vi "FlexMag - 24-03-2023.vi"() -> ()   [LabVIEW 2018] (continued)
                          n13249 = Not(x=w18358) -> (.not. x?=w18359:bool)
                        }
                      }
                    }
                  }
                  frame #13 {
                    n13250 = local write "TC2_speed_coefficient_set"(TRUE ("TC1_close_loop_set")) -> ()
                  }
                  frame #14 {
                    n13251 = flat-sequence {
                      frame #0 {
                        n13252 = local read "waiting_TC"() -> (w18362:u32)
                        n13253 = Wait (ms)(milliseconds to wait=w18362) -> ()  [unwired: 1 out]
                      }
                      frame #1 {
                        n13254 = while {
                          stop <- w18363 stop-if-true
                          n13255 = local read "TC2_speed_coefficient_set"() -> (w18364:bool)
                          n13256 = Wait Until Next ms Multiple(millisecond multiple=u32 300) -> ()  [unwired: 1 out]
                          n13257 = Not(x=w18364) -> (.not. x?=w18363:bool)
                        }
                      }
                    }
                  }
                  frame #15 {
                    n13258 = local write "TC2_AO1_polarity(pos_to_neg)"(TRUE ("TC1_close_loop_set")) -> ()
                  }
                  frame #16 {
                    n13259 = flat-sequence {
                      frame #0 {
                        n13260 = local read "waiting_TC"() -> (w18367:u32)
                        n13261 = Wait (ms)(milliseconds to wait=w18367) -> ()  [unwired: 1 out]
                      }
                      frame #1 {
                        n13262 = while {
                          stop <- w18369 stop-if-true
                          n13263 = local read "TC2_AO1_polarity(pos_to_neg)"() -> (w18368:bool)
                          n13264 = Wait Until Next ms Multiple(millisecond multiple=u32 300) -> ()  [unwired: 1 out]
                          n13265 = Not(x=w18368) -> (.not. x?=w18369:bool)
                        }
                      }
                    }
                  }
                  frame #17 {
                    n13266 = local write "TC1_AO1_upper_limit_set"(TRUE ("TC1_close_loop_set")) -> ()
                  }
                  frame #18 {
                    n13267 = flat-sequence {
                      frame #0 {
                        n13268 = local read "waiting_TC"() -> (w18372:u32)
                        n13269 = Wait (ms)(milliseconds to wait=w18372) -> ()  [unwired: 1 out]
                      }
                      frame #1 {
                        n13270 = while {
                          stop <- w18373 stop-if-true
                          n13271 = local read "TC1_AO1_upper_limit_set"() -> (w18374:bool)
                          n13272 = Wait Until Next ms Multiple(millisecond multiple=u32 300) -> ()  [unwired: 1 out]
                          n13273 = Not(x=w18374) -> (.not. x?=w18373:bool)
                        }
                      }
                    }
                  }
                  frame #19 {
                    n13274 = local write "TC1_AO1_bottom_limit_set"(TRUE ("TC1_close_loop_set")) -> ()
                  }
                  frame #20 {
                    n13275 = flat-sequence {
                      frame #0 {
                        n13276 = local read "waiting_TC"() -> (w18377:u32)
                        n13277 = Wait (ms)(milliseconds to wait=w18377) -> ()  [unwired: 1 out]
                      }
                      frame #1 {
                        n13278 = while {
                          stop <- w18379 stop-if-true
                          n13279 = local read "TC1_AO1_bottom_limit_set"() -> (w18378:bool)
                          n13280 = Wait Until Next ms Multiple(millisecond multiple=u32 300) -> ()  [unwired: 1 out]
                          n13281 = Not(x=w18378) -> (.not. x?=w18379:bool)
                        }
                      }
                    }
                  }
                  frame #21 {
                    n13282 = local write "TC2_AO1_upper_limit_set"(TRUE ("TC1_close_loop_set")) -> ()
                  }
                  frame #22 {
                    n13283 = flat-sequence {
                      frame #0 {
                        n13284 = local read "waiting_TC"() -> (w18382:u32)
                        n13285 = Wait (ms)(milliseconds to wait=w18382) -> ()  [unwired: 1 out]
                      }
                      frame #1 {
                        n13286 = while {
                          stop <- w18383 stop-if-true
                          n13287 = local read "TC2_AO1_upper_limit_set"() -> (w18384:bool)
                          n13288 = Wait Until Next ms Multiple(millisecond multiple=u32 300) -> ()  [unwired: 1 out]
                          n13289 = Not(x=w18384) -> (.not. x?=w18383:bool)
                        }
                      }
                    }
                  }
                  frame #23 {
                    n13290 = local write "TC2_AO1_bottom_limit_set"(TRUE ("TC1_close_loop_set")) -> ()
                  }
                  frame #24 {
                    n13291 = flat-sequence {
                      frame #0 {
                        n13292 = local read "waiting_TC"() -> (w18387:u32)
                        n13293 = Wait (ms)(milliseconds to wait=w18387) -> ()  [unwired: 1 out]
                      }
                      frame #1 {
                        n13294 = while {
                          stop <- w18389 stop-if-true
                          n13295 = local read "TC2_AO1_bottom_limit_set"() -> (w18388:bool)
                          n13296 = Wait Until Next ms Multiple(millisecond multiple=u32 300) -> ()  [unwired: 1 out]
                          n13297 = Not(x=w18388) -> (.not. x?=w18389:bool)
                        }
                      }
                    }
                  }
                  frame #25 {
                    n13298 = local write "TC1_regulation_type_selection"(TRUE ("TC1_regulation_type_selection")) -> ()
                  }
                  frame #26 {
                    n13299 = flat-sequence {
                      frame #0 {
                        n13300 = local read "waiting_TC"() -> (w18392:u32)
                        n13301 = Wait (ms)(milliseconds to wait=w18392) -> ()  [unwired: 1 out]
                      }
                      frame #1 {
                        n13302 = while {
                          stop <- w18393 stop-if-true
                          n13303 = local read "TC1_regulation_type_selection"() -> (w18394:bool)
                          n13304 = Wait Until Next ms Multiple(millisecond multiple=u32 300) -> ()  [unwired: 1 out]
                          n13305 = Not(x=w18394) -> (.not. x?=w18393:bool)
                        }
                      }
                    }
                  }
                  frame #27 {
                    n13306 = local write "TC2_regulation_type_selection"(TRUE ("TC2_regulation_type_selection")) -> ()
                  }
                  frame #28 {
                    n13307 = flat-sequence {
                      frame #0 {
                        n13308 = local read "waiting_TC"() -> (w18397:u32)
                        n13309 = Wait (ms)(milliseconds to wait=w18397) -> ()  [unwired: 1 out]
                      }
                      frame #1 {
                        n13310 = while {
                          stop <- w18399 stop-if-true
                          n13311 = local read "TC2_regulation_type_selection"() -> (w18398:bool)
                          n13312 = Wait Until Next ms Multiple(millisecond multiple=u32 300) -> ()  [unwired: 1 out]
                          n13313 = Not(x=w18398) -> (.not. x?=w18399:bool)
                        }
                      }
                    }
                  }
                  frame #29 {
                    n13314 = local write "TC2_setpoint_type"(TRUE ("TC2_setpoint_type")) -> ()
                  }
                  frame #30 {
                    n13315 = flat-sequence {
                      frame #0 {
                        n13316 = local read "waiting_TC"() -> (w18402:u32)
                        n13317 = Wait (ms)(milliseconds to wait=w18402) -> ()  [unwired: 1 out]
                      }
                      frame #1 {
                        n13318 = while {
                          stop <- w18403 stop-if-true
                          n13319 = local read "TC2_setpoint_type"() -> (w18404:bool)
                          n13320 = Wait Until Next ms Multiple(millisecond multiple=u32 300) -> ()  [unwired: 1 out]
                          n13321 = Not(x=w18404) -> (.not. x?=w18403:bool)
                        }
                      }
                    }
                  }
                  frame #31 {
                    n13322 = local write "TC1_setpoint_type"(TRUE ("TC1_setpoint_type")) -> ()
                  }
                  frame #32 {
                    n13323 = flat-sequence {
                      frame #0 {
                        n13324 = local read "waiting_TC"() -> (w18407:u32)
                        n13325 = Wait (ms)(milliseconds to wait=w18407) -> ()  [unwired: 1 out]
                      }
                      frame #1 {
                        n13326 = while {
                          stop <- w18409 stop-if-true
                          n13327 = local read "TC1_setpoint_type"() -> (w18408:bool)
                          n13328 = Wait Until Next ms Multiple(millisecond multiple=u32 300) -> ()  [unwired: 1 out]
                          n13329 = Not(x=w18408) -> (.not. x?=w18409:bool)
                        }
                      }
                    }
                  }
                  frame #33 {
                    n13330 = local write "TC parameter set"(FALSE ("TC parameter set")) -> ()
                  }
                }
              }
              frame True {
                n13331 = stacked-sequence {
                  frame #0 {
                    n13332 = local write "TC1_close_loop_coefficient"(sgl 100.0 ("TC1_close_loop_coefficient")) -> ()
                    n13333 = local write "TC1_speed_gain_value"(sgl 0.0 ("TC1_speed_gain_value")) -> ()
                    n13334 = local write "TC1_speed_coefficient_value"(sgl 0.0 ("TC1_speed_coefficient_value")) -> ()
                    n13335 = local write "TC1_AO1_upper_limit_value"(sgl 10.0 ("TC1_speed_coefficient_value")) -> ()
                    n13336 = local write "TC1_AO1_bottom_limit_value"(sgl 0.0 ("TC1_speed_coefficient_value")) -> ()
                    n13337 = local write "TC1_regulation_type_value"(sgl 1.0 ("TC1_speed_coefficient_value")) -> ()
                    n13338 = local write "TC1_setpoint_type_value"(sgl 0.0 ("TC1_speed_coefficient_value")) -> ()
                    n13339 = Wait (ms)(milliseconds to wait=u32 100) -> ()  [unwired: 1 out]
                    n13340 = local write "TC2_close_loop_coefficient"(sgl 0.0 ("TC2_close_loop_coefficient")) -> ()
                    n13341 = local write "TC2_speed_gain_value"(sgl 0.0 ("TC2_speed_gain_value")) -> ()
                    n13342 = local write "TC2_speed_coefficient_value"(sgl 100.0 ("TC2_speed_coefficient_value")) -> ()
                    n13343 = local write "TC2_AO1_upper_limit_value"(sgl 10.0 ("TC2_speed_gain_value")) -> ()
                    n13344 = local write "TC2_AO1_bottom_limit_value"(sgl 0.0 ("TC2_speed_coefficient_value")) -> ()
                    n13345 = local write "TC2_regulation_type_value"(sgl 0.0 ("TC2_speed_coefficient_value")) -> ()
                    n13346 = local write "TC2_setpoint_type_value"(sgl 0.0 ("TC2_speed_coefficient_value")) -> ()
                  }
                  frame #1 {
                    n13347 = local write "TC1_close_loop_set"(TRUE ("TC1_close_loop_set")) -> ()
                  }
                  frame #2 {
                    n13348 = flat-sequence {
                      frame #0 {
                        n13349 = local read "waiting_TC"() -> (w18428:u32)
                        n13350 = Wait (ms)(milliseconds to wait=w18428) -> ()  [unwired: 1 out]
                      }
                      frame #1 {
                        n13351 = while {
                          stop <- w18429 stop-if-true
                          n13352 = local read "TC1_close_loop_set"() -> (w18430:bool)
                          n13353 = Wait Until Next ms Multiple(millisecond multiple=u32 300) -> ()  [unwired: 1 out]
                          n13354 = Not(x=w18430) -> (.not. x?=w18429:bool)
                        }
                      }
                    }
                  }
                  frame #3 {
                    n13355 = local write "TC1_speed_gain_set"(TRUE ("TC1_close_loop_set")) -> ()
                  }
                  frame #4 {
                    n13356 = flat-sequence {
                      frame #0 {
                        n13357 = local read "waiting_TC"() -> (w18433:u32)
                        n13358 = Wait (ms)(milliseconds to wait=w18433) -> ()  [unwired: 1 out]
                      }
                      frame #1 {
                        n13359 = while {
                          stop <- w18435 stop-if-true
                          n13360 = local read "TC1_speed_gain_set"() -> (w18434:bool)
                          n13361 = Wait Until Next ms Multiple(millisecond multiple=u32 300) -> ()  [unwired: 1 out]
                          n13362 = Not(x=w18434) -> (.not. x?=w18435:bool)
                        }
                      }
                    }
                  }
                  frame #5 {
                    n13363 = local write "TC1_speed_coefficient_set"(TRUE ("TC1_close_loop_set")) -> ()
                  }
                  frame #6 {
                    n13364 = flat-sequence {
                      frame #0 {
                        n13365 = local read "waiting_TC"() -> (w18438:u32)
                        n13366 = Wait (ms)(milliseconds to wait=w18438) -> ()  [unwired: 1 out]
                      }
                      frame #1 {
                        n13367 = while {
                          stop <- w18439 stop-if-true
                          n13368 = local read "TC1_speed_coefficient_set"() -> (w18440:bool)
                          n13369 = Wait Until Next ms Multiple(millisecond multiple=u32 300) -> ()  [unwired: 1 out]
                          n13370 = Not(x=w18440) -> (.not. x?=w18439:bool)
                        }
                      }
                    }
                  }
                  frame #7 {
                    n13371 = local write "TC1_AO1_polarity(pos_to_neg)"(TRUE ("TC1_close_loop_set")) -> ()
                  }
                  frame #8 {
                    n13372 = flat-sequence {
                      frame #0 {
                        n13373 = local read "waiting_TC"() -> (w18443:u32)
                        n13374 = Wait (ms)(milliseconds to wait=w18443) -> ()  [unwired: 1 out]
                      }
                      frame #1 {
                        n13375 = while {
                          stop <- w18445 stop-if-true
                          n13376 = local read "TC1_AO1_polarity(pos_to_neg)"() -> (w18444:bool)
                          n13377 = Wait Until Next ms Multiple(millisecond multiple=u32 300) -> ()  [unwired: 1 out]
                          n13378 = Not(x=w18444) -> (.not. x?=w18445:bool)
                        }
                      }
                    }
                  }
                  frame #9 {
                    n13379 = local write "TC2_close_loop_set"(TRUE ("TC1_close_loop_set")) -> ()
                  }
                  frame #10 {
                    n13380 = flat-sequence {
                      frame #0 {
                        n13381 = local read "waiting_TC"() -> (w18448:u32)
                        n13382 = Wait (ms)(milliseconds to wait=w18448) -> ()  [unwired: 1 out]
                      }
                      frame #1 {
                        n13383 = while {
                          stop <- w18449 stop-if-true
                          n13384 = local read "TC2_close_loop_set"() -> (w18450:bool)
                          n13385 = Wait Until Next ms Multiple(millisecond multiple=u32 300) -> ()  [unwired: 1 out]
                          n13386 = Not(x=w18450) -> (.not. x?=w18449:bool)
                        }
                      }
                    }
                  }
                  frame #11 {
                    n13387 = local write "TC2_speed_gain_set"(TRUE ("TC1_close_loop_set")) -> ()
                  }
                  frame #12 {
                    n13388 = flat-sequence {
                      frame #0 {
                        n13389 = local read "waiting_TC"() -> (w18453:u32)
                        n13390 = Wait (ms)(milliseconds to wait=w18453) -> ()  [unwired: 1 out]
                      }
                      frame #1 {
                        n13391 = while {
                          stop <- w18455 stop-if-true
                          n13392 = local read "TC2_speed_gain_set"() -> (w18454:bool)
                          n13393 = Wait Until Next ms Multiple(millisecond multiple=u32 300) -> ()  [unwired: 1 out]
                          n13394 = Not(x=w18454) -> (.not. x?=w18455:bool)
                        }
                      }
                    }
                  }
                  frame #13 {
                    n13395 = local write "TC2_speed_coefficient_set"(TRUE ("TC1_close_loop_set")) -> ()
                  }
                  frame #14 {
                    n13396 = flat-sequence {
                      frame #0 {
                        n13397 = local read "waiting_TC"() -> (w18458:u32)
                        n13398 = Wait (ms)(milliseconds to wait=w18458) -> ()  [unwired: 1 out]
                      }
                      frame #1 {
                        n13399 = while {
                          stop <- w18459 stop-if-true
                          n13400 = local read "TC2_speed_coefficient_set"() -> (w18460:bool)
                          n13401 = Wait Until Next ms Multiple(millisecond multiple=u32 300) -> ()  [unwired: 1 out]
                          n13402 = Not(x=w18460) -> (.not. x?=w18459:bool)
                        }
                      }
                    }
                  }
                  frame #15 {
                    n13403 = local write "TC2_AO1_polarity(neg_to_pos)"(TRUE ("TC1_close_loop_set")) -> ()
                  }
                  frame #16 {
                    n13404 = flat-sequence {
                      frame #0 {
                        n13405 = local read "waiting_TC"() -> (w18463:u32)
                        n13406 = Wait (ms)(milliseconds to wait=w18463) -> ()  [unwired: 1 out]
                      }
                      frame #1 {
                        n13407 = while {
                          stop <- w18465 stop-if-true
                          n13408 = local read "TC2_AO1_polarity(neg_to_pos)"() -> (w18464:bool)
                          n13409 = Wait Until Next ms Multiple(millisecond multiple=u32 300) -> ()  [unwired: 1 out]
                          n13410 = Not(x=w18464) -> (.not. x?=w18465:bool)
                        }
                      }
                    }
                  }
                  frame #17 {
                    n13411 = local write "TC1_AO1_upper_limit_set"(TRUE ("TC1_close_loop_set")) -> ()
                  }
                  frame #18 {
                    n13412 = flat-sequence {
                      frame #0 {
                        n13413 = local read "waiting_TC"() -> (w18468:u32)
                        n13414 = Wait (ms)(milliseconds to wait=w18468) -> ()  [unwired: 1 out]
                      }
                      frame #1 {
                        n13415 = while {
                          stop <- w18469 stop-if-true
                          n13416 = local read "TC1_AO1_upper_limit_set"() -> (w18470:bool)
                          n13417 = Wait Until Next ms Multiple(millisecond multiple=u32 300) -> ()  [unwired: 1 out]
                          n13418 = Not(x=w18470) -> (.not. x?=w18469:bool)
                        }
                      }
                    }
                  }
                  frame #19 {
                    n13419 = local write "TC1_AO1_bottom_limit_set"(TRUE ("TC1_close_loop_set")) -> ()
                  }
                  frame #20 {
                    n13420 = flat-sequence {
                      frame #0 {
                        n13421 = local read "waiting_TC"() -> (w18473:u32)
                        n13422 = Wait (ms)(milliseconds to wait=w18473) -> ()  [unwired: 1 out]
                      }
                      frame #1 {
                        n13423 = while {
                          stop <- w18475 stop-if-true
                          n13424 = local read "TC1_AO1_bottom_limit_set"() -> (w18474:bool)
                          n13425 = Wait Until Next ms Multiple(millisecond multiple=u32 300) -> ()  [unwired: 1 out]
                          n13426 = Not(x=w18474) -> (.not. x?=w18475:bool)
                        }
                      }
                    }
                  }
                  frame #21 {
                    n13427 = local write "TC2_AO1_upper_limit_set"(TRUE ("TC1_close_loop_set")) -> ()
                  }
                  frame #22 {
                    n13428 = flat-sequence {
                      frame #0 {
                        n13429 = local read "waiting_TC"() -> (w18478:u32)
                        n13430 = Wait (ms)(milliseconds to wait=w18478) -> ()  [unwired: 1 out]
                      }
                      frame #1 {
                        n13431 = while {
                          stop <- w18479 stop-if-true
                          n13432 = local read "TC2_AO1_upper_limit_set"() -> (w18480:bool)
                          n13433 = Wait Until Next ms Multiple(millisecond multiple=u32 300) -> ()  [unwired: 1 out]
                          n13434 = Not(x=w18480) -> (.not. x?=w18479:bool)
                        }
                      }
                    }
                  }
                  frame #23 {
                    n13435 = local write "TC2_AO1_bottom_limit_set"(TRUE ("TC1_close_loop_set")) -> ()
                  }
                  frame #24 {
                    n13436 = flat-sequence {
                      frame #0 {
                        n13437 = local read "waiting_TC"() -> (w18483:u32)
                        n13438 = Wait (ms)(milliseconds to wait=w18483) -> ()  [unwired: 1 out]
                      }
                      frame #1 {
                        n13439 = while {
                          stop <- w18485 stop-if-true
                          n13440 = local read "TC2_AO1_bottom_limit_set"() -> (w18484:bool)
                          n13441 = Wait Until Next ms Multiple(millisecond multiple=u32 300) -> ()  [unwired: 1 out]
                          n13442 = Not(x=w18484) -> (.not. x?=w18485:bool)
                        }
                      }
                    }
                  }
                  frame #25 {
                    n13443 = local write "TC1_regulation_type_selection"(TRUE ("TC1_close_loop_set")) -> ()
                  }
                  frame #26 {
                    n13444 = flat-sequence {
                      frame #0 {
                        n13445 = local read "waiting_TC"() -> (w18488:u32)
                        n13446 = Wait (ms)(milliseconds to wait=w18488) -> ()  [unwired: 1 out]
                      }
                      frame #1 {
                        n13447 = while {
                          stop <- w18489 stop-if-true
                          n13448 = local read "TC1_regulation_type_selection"() -> (w18490:bool)
                          n13449 = Wait Until Next ms Multiple(millisecond multiple=u32 300) -> ()  [unwired: 1 out]
                          n13450 = Not(x=w18490) -> (.not. x?=w18489:bool)
                        }
                      }
                    }
                  }
                  frame #27 {
                    n13451 = local write "TC2_regulation_type_selection"(TRUE ("TC1_close_loop_set")) -> ()
                  }
                  frame #28 {
                    n13452 = flat-sequence {
                      frame #0 {
                        n13453 = local read "waiting_TC"() -> (w18493:u32)
                        n13454 = Wait (ms)(milliseconds to wait=w18493) -> ()  [unwired: 1 out]
                      }
                      frame #1 {
                        n13455 = while {
                          stop <- w18495 stop-if-true
                          n13456 = local read "TC2_regulation_type_selection"() -> (w18494:bool)
                          n13457 = Wait Until Next ms Multiple(millisecond multiple=u32 300) -> ()  [unwired: 1 out]
                          n13458 = Not(x=w18494) -> (.not. x?=w18495:bool)
                        }
                      }
                    }
                  }
                  frame #29 {
                    n13459 = local write "TC1_setpoint_type"(TRUE ("TC1_setpoint_type")) -> ()
                  }
                  frame #30 {
                    n13460 = flat-sequence {
                      frame #0 {
                        n13461 = local read "waiting_TC"() -> (w18498:u32)
                        n13462 = Wait (ms)(milliseconds to wait=w18498) -> ()  [unwired: 1 out]
                      }
                      frame #1 {
                        n13463 = while {
                          stop <- w18499 stop-if-true
                          n13464 = local read "TC1_setpoint_type"() -> (w18500:bool)
                          n13465 = Wait Until Next ms Multiple(millisecond multiple=u32 300) -> ()  [unwired: 1 out]
                          n13466 = Not(x=w18500) -> (.not. x?=w18499:bool)
                        }
                      }
                    }
                  }
                  frame #31 {
                    n13467 = local write "TC2_setpoint_type"(TRUE ("TC2_setpoint_type")) -> ()
                  }
                  frame #32 {
                    n13468 = flat-sequence {
                      frame #0 {
                        n13469 = local read "waiting_TC"() -> (w18503:u32)
                        n13470 = Wait (ms)(milliseconds to wait=w18503) -> ()  [unwired: 1 out]
                      }
                      frame #1 {
                        n13471 = while {
                          stop <- w18505 stop-if-true
                          n13472 = local read "TC2_setpoint_type"() -> (w18504:bool)
                          n13473 = Wait Until Next ms Multiple(millisecond multiple=u32 300) -> ()  [unwired: 1 out]
                          n13474 = Not(x=w18504) -> (.not. x?=w18505:bool)
                        }
                      }
                    }
                  }
                  frame #33 {
                    n13475 = local write "TC parameter set"(FALSE ("TC parameter set")) -> ()
                  }
                }
              }
            }
          }
          frame True {
            n13476 = local write "TC parameter set"(FALSE ("TC parameter set")) -> ()
          }
        }
        n13477 = local write "parameters led"(TRUE) -> ()
      }
    }
  }
  n13478 = while {
    stop <- FALSE stop-if-true
    n13479 = Wait Until Next ms Multiple(millisecond multiple=u32 300) -> ()  [unwired: 1 out]
    n13480 = case shown="True" "cycle roll stop" {
      frame False {
      }
      frame True {
        n13481 = stacked-sequence {
          frame #0 {
            w18519 = FALSE
            w18520 = FALSE
            n13482 = local write "CH1_Motor DO"(w18520) -> ()
            n13483 = local write "CH2_Motor DO"(w18520) -> ()
            n13484 = local write "CH3_Motor DO"(w18520) -> ()
            n13485 = local write "CH4_Motor DO"(w18520) -> ()
            n13486 = local write "forward roll"(w18519) -> ()
            n13487 = local write "back roll"(w18519) -> ()
            n13488 = local write "position"(w18519) -> ()
            n13489 = local write "cycle roll start"(FALSE) -> ()
            n13490 = Wait (ms)(milliseconds to wait=u32 1000) -> ()  [unwired: 1 out]
          }
          frame #1 {
            n13491 = local write "cycle roll stop"(FALSE ("stop roll")) -> ()
          }
        }
      }
    }
    n13492 = case shown="True" "stop roll" {
      frame False {
      }
      frame True {
        n13493 = stacked-sequence {
          frame #0 {
            w18514 = FALSE
            w18515 = FALSE
            n13494 = local write "CH1_Motor DO"(w18515) -> ()
            n13495 = local write "CH2_Motor DO"(w18515) -> ()
            n13496 = local write "CH3_Motor DO"(w18515) -> ()
            n13497 = local write "CH4_Motor DO"(w18515) -> ()
            n13498 = local write "forward roll"(w18514) -> ()
            n13499 = local write "back roll"(w18514) -> ()
            n13500 = local write "position"(w18514) -> ()
            n13501 = Wait (ms)(milliseconds to wait=u32 1000) -> ()  [unwired: 1 out]
          }
          frame #1 {
            n13502 = local write "stop roll"(FALSE ("stop roll")) -> ()
          }
        }
      }
    }
  }
  n13503 = while {
    stop <- FALSE stop-if-true
    n13504 = Wait Until Next ms Multiple(millisecond multiple=u32 300) -> ()  [unwired: 1 out]
    n13505 = Build Array(FALSE ("element"), "ch1 pd clear", "ch2 pd clear", "ch3 pd clear", "ch4 pd clear", "ch1 sd clear", "ch2 sd clear", "ch3 sd clear", "ch4 sd clear", "trns clear", "coating clear") -> (w18534:bool[])
    n13506 = Boolean Array To Number(Boolean array=w18534) -> (number=w18535:u32)
    n13507 = Mantissa & Exponent(0:w18535) -> (2:w18533:dbl)  [unwired: 1 out]
    n13508 = case shown="1" w18533 {
      frame 0, Default {
      }
      frame 1 {
        w18538 = FALSE ("ch1 atms close led")
        n13509 = local write "ch1 pd clear"(w18538) -> ()
        "ch1 atms close led" <- w18538
        "ch1 ch vbv close led" <- w18538
        "ch1 pl vbv close led" <- w18538
        "ch1 tp bv open led" <- w18538
        "ch1 pc gv open led" <- w18538
        "ch1 mp start led" <- w18538
        "ch1 trns bp left close led" <- w18538
        "ch1-ch2 trns gv close led 2" <- w18538
        "ch1 pl press under 0.05 T led" <- w18538
        "ch1 ch press under 0.5 T led" <- w18538
        "ch1 tp start led" <- w18538
        "ch1 trns bp left open led" <- w18538
        "ch1 ch press under 0.01 T led" <- w18538
        "ch1 cc open led" <- w18538
        "ch1 desired pressure led" <- w18538
        "ch1 pd completed led" <- w18538
      }
      frame 2 {
        w18539 = FALSE ("ch1 atms close led")
        n13510 = local write "ch2 pd clear"(w18539) -> ()
        "ch2 atms close led" <- w18539
        "ch2 ch vbv close led" <- w18539
        "ch2 pl vbv close led" <- w18539
        "ch2 tp bv open led" <- w18539
        "ch2 pc gv open led" <- w18539
        "ch2 mp start led" <- w18539
        "ch2 trns bp left close led" <- w18539
        "ch1-ch2 trns gv close led" <- w18539
        "ch2 pl press under 0.05 T led" <- w18539
        "ch2 ch press under 0.5 T led" <- w18539
        "ch2 tp start led" <- w18539
        "ch2 trns bp left open led" <- w18539
        "ch2 ch press under 0.01 T led" <- w18539
        "ch2 cc open led" <- w18539
        "ch2 desired pressure led" <- w18539
        "ch2 pd completed led" <- w18539
        "ch2 trns bp right close led" <- w18539
        "ch2 trns bp right open led" <- w18539
        "ch2-ch3 trns gv close led" <- w18539
      }
      frame 3 {
        w18540 = FALSE ("ch1 atms close led")
        n13511 = local write "ch3 pd clear"(w18540) -> ()
        "ch3 atms close led" <- w18540
        "ch3 ch vbv close led" <- w18540
        "ch3 pl vbv close led" <- w18540
        "ch3 tp bv open led" <- w18540
        "ch3 pc gv open led" <- w18540
        "ch3 mp start led" <- w18540
        "ch3 trns bp left close led" <- w18540
        "ch3-ch2 trns gv close led" <- w18540
        "ch3 pl press under 0.05 T led" <- w18540
        "ch3 ch press under 0.5 T led" <- w18540
        "ch3 tp start led" <- w18540
        "ch3 trns bp left open led" <- w18540
        "ch3 ch press under 0.01 T led" <- w18540
        "ch3 cc open led" <- w18540
        "ch3 desired pressure led" <- w18540
        "ch3 pd completed led" <- w18540
        "ch3 trns bp right close led" <- w18540
        "ch3 trns bp right open led" <- w18540
        "ch3-ch4 trns gv close led" <- w18540
      }
      frame 4 {
        w18541 = FALSE ("ch1 atms close led")
        n13512 = local write "ch4 pd clear"(w18541) -> ()
        "ch4 atms close led" <- w18541
        "ch4 ch vbv close led" <- w18541
        "ch4 pl vbv close led" <- w18541
        "ch4 tp bv open led" <- w18541
        "ch4 pc gv open led" <- w18541
        "ch4 mp start led" <- w18541
        "ch4 pl press under 0.05 T led" <- w18541
        "ch4 ch press under 0.5 T led" <- w18541
        "ch4 tp start led" <- w18541
        "ch4 ch press under 0.01 T led" <- w18541
        "ch4 cc open led" <- w18541
        "ch4 desired pressure led" <- w18541
        "ch4 pd completed led" <- w18541
        "ch4 trns bp right close led" <- w18541
        "ch4 trns bp right open led" <- w18541
        "ch4-ch3 trns gv close led" <- w18541
      }
      frame 5 {
        w18542 = FALSE ("ch1 atms close led")
        n13513 = local write "ch1 sd clear"(w18542) -> ()
        "ch1 sd cc close led" <- w18542
        "ch1 sd tp stop led" <- w18542
        "ch1 sd bg bv close led" <- w18542
        "ch1 sd mp stop led" <- w18542
        "ch1 sd pl vbv open led" <- w18542
        "ch1 sd pcgv open led" <- w18542
        "ch1 sd tp bv close led" <- w18542
        "ch1 sd atms close led" <- w18542
        "ch1 sd pcgv close led" <- w18542
        "ch1 sd trns bp left open led" <- w18542
        "ch1 sd ch vbv open led" <- w18542
        "ch1 sd trns bp left close led" <- w18542
        "ch1 sd PL atm on led" <- w18542
        "ch1 sd PL-CH atm on led" <- w18542
        "ch1 sd completed led" <- w18542
      }
      frame 6 {
        w18543 = FALSE ("ch1 atms close led")
        n13514 = local write "ch2 sd clear"(w18543) -> ()
        "ch2 sd cc close led" <- w18543
        "ch2 sd tp stop led" <- w18543
        "ch2 sd bg bv close led" <- w18543
        "ch2 sd mp stop led" <- w18543
        "ch2 sd pl vbv open led" <- w18543
        "ch2 sd pcgv open led" <- w18543
        "ch2 sd tp bv close led" <- w18543
        "ch2 sd atms close led" <- w18543
        "ch2 sd pcgv close led" <- w18543
        "ch2 sd trns bp left open led" <- w18543
        "ch2 sd ch vbv open led" <- w18543
        "ch2 sd trns bp left close led" <- w18543
        "ch2 sd PL atm on led" <- w18543
        "ch2 sd PL-CH atm on led" <- w18543
        "ch2 sd completed led" <- w18543
        "ch2 sd trns bp right open led" <- w18543
        "ch2 sd trns bp right close led" <- w18543
      }
      frame 7 {
        w18544 = FALSE ("ch1 atms close led")
        n13515 = local write "ch3 sd clear"(w18544) -> ()
        "ch3 sd cc close led" <- w18544
        "ch3 sd tp stop led" <- w18544
        "ch3 sd bg bv close led" <- w18544
        "ch3 sd mp stop led" <- w18544
        "ch3 sd pl vbv open led" <- w18544
        "ch3 sd pcgv open led" <- w18544
        "ch3 sd tp bv close led" <- w18544
        "ch3 sd atms close led" <- w18544
        "ch3 sd pcgv close led" <- w18544
        "ch3 sd trns bp left open led" <- w18544
        "ch3 sd ch vbv open led" <- w18544
        "ch3 sd trns bp left close led" <- w18544
        "ch3 sd PL atm on led" <- w18544
        "ch3 sd PL-CH atm on led" <- w18544
        "ch3 sd completed led" <- w18544
        "ch3 sd trns bp right open led" <- w18544
        "ch3 sd trns bp right close led" <- w18544
      }
      frame 8 {
        w18545 = FALSE ("ch1 atms close led")
        n13516 = local write "ch4 sd clear"(w18545) -> ()
        "ch4 sd cc close led" <- w18545
        "ch4 sd tp stop led" <- w18545
        "ch4 sd bg bv close led" <- w18545
        "ch4 sd mp stop led" <- w18545
        "ch4 sd pl vbv open led" <- w18545
        "ch4 sd pcgv open led" <- w18545
        "ch4 sd tp bv close led" <- w18545
        "ch4 sd atms close led" <- w18545
        "ch4 sd pcgv close led" <- w18545
        "ch4 sd trns bp right open led" <- w18545
        "ch4 sd ch vbv open led" <- w18545
        "ch4 sd trns bp right close led" <- w18545
        "ch4 sd PL atm on led" <- w18545
        "ch4 sd PL-CH atm on led" <- w18545
        "ch4 sd completed led" <- w18545
      }
      frame 9 {
        n13517 = stacked-sequence {
          frame #0 {
            w18546 = FALSE ("element")
            n13518 = local write "trns clear"(w18546) -> ()
            "trns pre check led 1" <- w18546
            "trns pre check led 2" <- w18546
            "trns pre check led 3" <- w18546
            "trns pre check led 4" <- w18546
            "trns pre check led 8" <- w18546
            "trns pre check led 7" <- w18546
            "trns pre check led 6" <- w18546
            "trns pre check led 5" <- w18546
            "trns pre check led 9" <- w18546
            "trns pre check led 10" <- w18546
            "trns pre check led 11" <- w18546
            "trns pre check led 12" <- w18546
          }
          frame #1 {
            w18547 = FALSE ("trns 1-2 led 19")
            w18548 = FALSE
            "trns 1-2 led 1" <- w18548
            "trns 1-2 led 2" <- w18548
            "trns 1-2 led 4" <- w18548
            "trns 1-2 led 3" <- w18548
            "trns 1-2 led 5" <- w18548
            "trns 1-2 led 6" <- w18548
            "trns 1-2 led 8" <- w18548
            "trns 1-2 led 7" <- w18548
            "trns 1-2 led 9" <- w18548
            "trns 1-2 led 10" <- w18548
            "trns 1-2 led 11" <- w18548
            "trns 1-2 led 12" <- w18548
            "trns 1-2 led 13" <- w18548
            "trns 1-2 led 14" <- w18548
            "trns 1-2 led 15" <- w18548
            "trns 1-2 led 16" <- w18548
            "trns 1-2 led 17" <- w18548
            "trns 1-2 led 18" <- w18548
            "trns 1-2 led 19" <- w18547
            "trns 1-2 led 20" <- w18547
            "trns 1-2 led 21" <- w18547
            "trns 1-2 led 22" <- w18547
            "trns 1-2 led 23" <- w18547
          }
          frame #2 {
            w18549 = FALSE
            w18550 = FALSE
            "trns 2-3 led 1" <- w18550
            "trns 2-3 led 2" <- w18550
            "trns 2-3 led 4" <- w18550
            "trns 2-3 led 3" <- w18550
            "trns 2-3 led 8" <- w18550
            "trns 2-3 led 7" <- w18550
            "trns 2-3 led 6" <- w18550
            "trns 2-3 led 5" <- w18550
            "trns 2-3 led 12" <- w18550
            "trns 2-3 led 11" <- w18550
            "trns 2-3 led 10" <- w18550
            "trns 2-3 led 9" <- w18550
            "trns 2-3 led 16" <- w18550
            "trns 2-3 led 15" <- w18550
            "trns 2-3 led 14" <- w18550
            "trns 2-3 led 13" <- w18550
            "trns 2-3 led 17" <- w18550
            "trns 2-3 led 18" <- w18550
            "trns 2-3 led 19" <- w18549
            "trns 2-3 led 20" <- w18549
            "trns 2-3 led 22" <- w18549
            "trns 2-3 led 21" <- w18549
            "trns 2-3 led 23" <- w18549
            "trns 2-3 led 24" <- w18549
          }
          frame #3 {
            w18551 = FALSE
            w18552 = FALSE
            "trns 3-4 led 1" <- w18552
            "trns 3-4 led 2" <- w18552
            "trns 3-4 led 4" <- w18552
            "trns 3-4 led 3" <- w18552
            "trns 3-4 led 8" <- w18552
            "trns 3-4 led 7" <- w18552
            "trns 3-4 led 6" <- w18552
            "trns 3-4 led 5" <- w18552
            "trns 3-4 led 12" <- w18552
            "trns 3-4 led 11" <- w18552
            "trns 3-4 led 10" <- w18552
            "trns 3-4 led 9" <- w18552
            "trns 3-4 led 16" <- w18552
            "trns 3-4 led 15" <- w18552
            "trns 3-4 led 14" <- w18552
            "trns 3-4 led 13" <- w18552
            "trns 3-4 led 17" <- w18552
            "trns 3-4 led 18" <- w18552
            "trns 3-4 led 19" <- w18551
            "trns 3-4 led 20" <- w18551
            "trns 3-4 led 22" <- w18551
            "trns 3-4 led 21" <- w18551
            "trns 3-4 led 23" <- w18551
            "trns 3-4 led 24" <- w18551
          }
          frame #4 {
            w18553 = FALSE
            w18554 = FALSE
            "trns 2-1 led 1" <- w18554
            "trns 2-1 led 2" <- w18554
            "trns 2-1 led 4" <- w18554
            "trns 2-1 led 3" <- w18554
            "trns 2-1 led 8" <- w18554
            "trns 2-1 led 7" <- w18554
            "trns 2-1 led 6" <- w18554
            "trns 2-1 led 5" <- w18554
            "trns 2-1 led 12" <- w18554
            "trns 2-1 led 11" <- w18554
            "trns 2-1 led 10" <- w18554
            "trns 2-1 led 9" <- w18554
            "trns 2-1 led 16" <- w18554
            "trns 2-1 led 15" <- w18554
            "trns 2-1 led 14" <- w18554
            "trns 2-1 led 13" <- w18554
            "trns 2-1 led 17" <- w18554
            "trns 2-1 led 18" <- w18554
            "trns 2-1 led 19" <- w18553
            "trns 2-1 led 20" <- w18553
            "trns 2-1 led 22" <- w18553
            "trns 2-1 led 21" <- w18553
            "trns 2-1 led 23" <- w18553
            "trns 2-1 led 24" <- w18553
          }
          frame #5 {
            w18555 = FALSE
            w18556 = FALSE
            "trns 3-2 led 1" <- w18556
            "trns 3-2 led 2" <- w18556
            "trns 3-2 led 4" <- w18556
            "trns 3-2 led 3" <- w18556
            "trns 3-2 led 8" <- w18556
            "trns 3-2 led 7" <- w18556
            "trns 3-2 led 6" <- w18556
            "trns 3-2 led 5" <- w18556
            "trns 3-2 led 12" <- w18556
            "trns 3-2 led 11" <- w18556
            "trns 3-2 led 10" <- w18556
            "trns 3-2 led 9" <- w18556
            "trns 3-2 led 16" <- w18556
            "trns 3-2 led 15" <- w18556
            "trns 3-2 led 14" <- w18556
            "trns 3-2 led 13" <- w18556
            "trns 3-2 led 17" <- w18556
            "trns 3-2 led 18" <- w18556
            "trns 3-2 led 19" <- w18555
            "trns 3-2 led 20" <- w18555
            "trns 3-2 led 22" <- w18555
            "trns 3-2 led 21" <- w18555
            "trns 3-2 led 23" <- w18555
            "trns 3-2 led 24" <- w18555
          }
          frame #6 {
            w18557 = FALSE
            w18558 = FALSE
            "trns 4-3 led 1" <- w18558
            "trns 4-3 led 2" <- w18558
            "trns 4-3 led 4" <- w18558
            "trns 4-3 led 3" <- w18558
            "trns 4-3 led 8" <- w18558
            "trns 4-3 led 7" <- w18558
            "trns 4-3 led 6" <- w18558
            "trns 4-3 led 5" <- w18558
            "trns 4-3 led 12" <- w18558
            "trns 4-3 led 11" <- w18558
            "trns 4-3 led 10" <- w18558
            "trns 4-3 led 9" <- w18558
            "trns 4-3 led 16" <- w18558
            "trns 4-3 led 15" <- w18558
            "trns 4-3 led 14" <- w18558
            "trns 4-3 led 13" <- w18558
            "trns 4-3 led 17" <- w18558
            "trns 4-3 led 18" <- w18558
            "trns 4-3 led 19" <- w18557
            "trns 4-3 led 20" <- w18557
            "trns 4-3 led 22" <- w18557
            "trns 4-3 led 21" <- w18557
            "trns 4-3 led 23" <- w18557
          }
        }
      }
      frame 10 {
        n13519 = stacked-sequence {
          frame #0 {
          }
          frame #1 {
            w18559 = FALSE ("coating ch2 led 17")
            w18560 = FALSE
            n13520 = local write "coating ch2 led 1"(w18560) -> ()
            n13521 = local write "coating ch2 led 2"(w18560) -> ()
            n13522 = local write "coating ch2 led 3"(w18560) -> ()
            n13523 = local write "coating ch2 led 4"(w18560) -> ()
            n13524 = local write "coating ch2 led 5"(w18560) -> ()
            n13525 = local write "coating ch2 led 6"(w18560) -> ()
            n13526 = local write "coating ch2 led 7"(w18560) -> ()
            n13527 = local write "coating ch2 led 8"(w18560) -> ()
            n13528 = local write "coating ch2 led 9"(w18560) -> ()
            n13529 = local write "coating ch2 led 10"(w18560) -> ()
            n13530 = local write "coating ch2 led 11"(w18560) -> ()
            n13531 = local write "coating ch2 led 12"(w18560) -> ()
            n13532 = local write "coating ch2 led 13"(w18560) -> ()
            n13533 = local write "coating ch2 led 14"(w18560) -> ()
            n13534 = local write "coating ch2 led 15"(w18560) -> ()
            n13535 = local write "coating ch2 led 16"(w18560) -> ()
            n13536 = local write "coating ch2 led 17"(w18559) -> ()
            n13537 = local write "coating ch2 led 18"(w18559) -> ()
            n13538 = local write "coating ch2 led 19"(w18559) -> ()
            n13539 = local write "coating ch2 led 20"(w18559) -> ()
          }
          frame #2 {
            w18561 = FALSE ("coating ch2 led 17")
            w18562 = FALSE
            n13540 = local write "coating ch3 led 1"(w18562) -> ()
            n13541 = local write "coating ch3 led 2"(w18562) -> ()
            n13542 = local write "coating ch3 led 3"(w18562) -> ()
            n13543 = local write "coating ch3 led 4"(w18562) -> ()
            n13544 = local write "coating ch3 led 5"(w18562) -> ()
            n13545 = local write "coating ch3 led 6"(w18562) -> ()
            n13546 = local write "coating ch3 led 7"(w18562) -> ()
            n13547 = local write "coating ch3 led 8"(w18562) -> ()
            n13548 = local write "coating ch3 led 9"(w18562) -> ()
            n13549 = local write "coating ch3 led 10"(w18562) -> ()
            n13550 = local write "coating ch3 led 11"(w18562) -> ()
            n13551 = local write "coating ch3 led 12"(w18562) -> ()
            n13552 = local write "coating ch3 led 13"(w18562) -> ()
            n13553 = local write "coating ch3 led 14"(w18562) -> ()
            n13554 = local write "coating ch3 led 15"(w18562) -> ()
            n13555 = local write "coating ch3 led 16"(w18562) -> ()
            n13556 = local write "coating ch3 led 17"(w18561) -> ()
            n13557 = local write "coating ch3 led 18"(w18561) -> ()
            n13558 = local write "coating ch3 led 19"(w18561) -> ()
            n13559 = local write "coating ch3 led 20"(w18561) -> ()
          }
          frame #3 {
            w18563 = FALSE ("coating ch2 led 17")
            w18564 = FALSE
            n13560 = local write "coating ch4 led 1"(w18564) -> ()
            n13561 = local write "coating ch4 led 2"(w18564) -> ()
            n13562 = local write "coating ch4 led 3"(w18564) -> ()
            n13563 = local write "coating ch4 led 4"(w18564) -> ()
            n13564 = local write "coating ch4 led 5"(w18564) -> ()
            n13565 = local write "coating ch4 led 6"(w18564) -> ()
            n13566 = local write "coating ch4 led 7"(w18564) -> ()
            n13567 = local write "coating ch4 led 8"(w18564) -> ()
            n13568 = local write "coating ch4 led 9"(w18564) -> ()
            n13569 = local write "coating ch4 led 10"(w18564) -> ()
            n13570 = local write "coating ch4 led 11"(w18564) -> ()
            n13571 = local write "coating ch4 led 12"(w18564) -> ()
            n13572 = local write "coating ch4 led 13"(w18564) -> ()
            n13573 = local write "coating ch4 led 14"(w18564) -> ()
            n13574 = local write "coating ch4 led 15"(w18564) -> ()
            n13575 = local write "coating ch4 led 16"(w18564) -> ()
            n13576 = local write "coating ch4 led 17"(w18563) -> ()
            n13577 = local write "coating ch4 led 18"(w18563) -> ()
            n13578 = local write "coating ch4 led 19"(w18563) -> ()
            n13579 = local write "coating ch4 led 20"(w18563) -> ()
          }
        }
      }
    }
  }
  n13580 = while {
    stop <- FALSE stop-if-true
    n13581 = Wait Until Next ms Multiple(millisecond multiple=u32 300) -> ()  [unwired: 1 out]
    n13582 = case shown="True" "cycle roll start" {
      frame False {
      }
      frame True {
        n13583 = stacked-sequence {
          frame #0 {
            n13584 = local read "step count"() -> (w18570:dbl)
            n13585 = local write "cycle step count"(w18570) -> ()
            n13586 = Wait (ms)(milliseconds to wait=u32 100) -> ()  [unwired: 1 out]
            "Remaining Cycle" <- "Number of Cycle"
          }
          frame #1 {
            n13587 = while {
              stop <- w18576 stop-if-true
              n13588 = local read "Remaining Cycle"() -> (w18577:u8)
              n13589 = local read "cycle roll stop"() -> (w18573:bool)
              n13590 = Wait Until Next ms Multiple(millisecond multiple=u32 300) -> ()  [unwired: 1 out]
              n13591 = Greater?(x=w18577, y=u8 0) -> (0:w18574:bool)
              n13592 = case shown="True" w18574 {
                frame False {
                }
                frame True {
                  n13593 = stacked-sequence {
                    frame #0 {
                      n13594 = local write "step count"("cycle step count") -> ()
                    }
                    frame #1 {
                      n13595 = local read "cycle roll start"() -> (w18579:bool)
                      n13596 = case shown="True" w18579 {
                        frame False {
                        }
                        frame True {
                          n13597 = local write "forward roll"(TRUE ("forward roll")) -> ()
                        }
                      }
                    }
                    frame #2 {
                      n13598 = local read "cycle roll start"() -> (w18581:bool)
                      n13599 = case shown="True" w18581 {
                        frame False {
                        }
                        frame True {
                          n13600 = Wait (ms)(milliseconds to wait=u32 500) -> ()  [unwired: 1 out]
                        }
                      }
                    }
                    frame #3 {
                      n13601 = while {
                        stop <- w18587 stop-if-true
                        n13602 = local read "cycle roll stop"() -> (w18584:bool)
                        n13603 = local read "forward roll"() -> (w18586:bool)
                        n13604 = Not(x=w18586) -> (.not. x?=w18585:bool)
                        n13605 = Or(x=w18585, y=w18584) -> (x .or. y?=w18587:bool)
                        n13606 = Wait Until Next ms Multiple(millisecond multiple=u32 300) -> ()  [unwired: 1 out]
                      }
                    }
                    frame #4 {
                      n13607 = local read "cycle roll start"() -> (w18588:bool)
                      n13608 = case shown="True" w18588 {
                        frame False {
                        }
                        frame True {
                          n13609 = local read "cycle step count"() -> (w18589:sgl)
                          n13610 = local write "step count"(w18589) -> ()
                          n13611 = Wait (ms)(milliseconds to wait=u32 5000) -> ()  [unwired: 1 out]
                        }
                      }
                    }
                    frame #5 {
                      n13612 = local read "cycle roll start"() -> (w18591:bool)
                      n13613 = case shown="True" w18591 {
                        frame False {
                        }
                        frame True {
                          n13614 = local write "back roll"(TRUE ("forward roll")) -> ()
                        }
                      }
                    }
                    frame #6 {
                      n13615 = local read "cycle roll start"() -> (w18593:bool)
                      n13616 = case shown="True" w18593 {
                        frame False {
                        }
                        frame True {
                          n13617 = Wait (ms)(milliseconds to wait=u32 500) -> ()  [unwired: 1 out]
                        }
                      }
                    }
                    frame #7 {
                      n13618 = while {
                        stop <- w18599 stop-if-true
                        n13619 = local read "cycle roll stop"() -> (w18596:bool)
                        n13620 = local read "back roll"() -> (w18598:bool)
                        n13621 = Not(x=w18598) -> (.not. x?=w18597:bool)
                        n13622 = Or(x=w18597, y=w18596) -> (x .or. y?=w18599:bool)
                        n13623 = Wait Until Next ms Multiple(millisecond multiple=u32 300) -> ()  [unwired: 1 out]
                      }
                    }
                    frame #8 {
                      n13624 = local read "cycle roll start"() -> (w18600:bool)
                      n13625 = case shown="True" w18600 {
                        frame False {
                        }
                        frame True {
                          n13626 = Wait (ms)(milliseconds to wait=u32 500) -> ()  [unwired: 1 out]
                        }
                      }
                    }
                    frame #9 {
                      n13627 = local read "cycle roll start"() -> (w18602:bool)
                      n13628 = case shown="True" w18602 {
                        frame False {
                        }
                        frame True {
                          n13629 = local read "Remaining Cycle"() -> (w18605:u8)
                          n13630 = Decrement(x=w18605) -> (x-1=w18604:u8)
                          n13631 = local write "Remaining Cycle"(w18604) -> ()
                          n13632 = Wait (ms)(milliseconds to wait=u32 200) -> ()  [unwired: 1 out]
                        }
                      }
                    }
                    frame #10 {
                      n13633 = local read "cycle roll start"() -> (w18606:bool)
                      n13634 = case shown="True" w18606 {
                        frame False {
                        }
                        frame True {
                          n13635 = Wait (ms)(milliseconds to wait=u32 200) -> ()  [unwired: 1 out]
                        }
                      }
                    }
                  }
                }
              }
              n13636 = Not(x=w18574) -> (.not. x?=w18575:bool)
              n13637 = Or(x=w18575, y=w18573) -> (x .or. y?=w18576:bool)
            }
          }
          frame #2 {
            n13638 = local write "cycle roll start"(FALSE ("cycle roll start")) -> ()
            n13639 = Wait (ms)(milliseconds to wait=u32 500) -> ()  [unwired: 1 out]
          }
        }
      }
    }
  }
  n13640 = while {
    stop <- FALSE stop-if-true
    # "12"
    # "11"
    # "10"
    # "9"
    # "8"
    # "7"
    # "6"
    # "5"
    # "4"
    # "3"
    # "2"
    # "1"
    n13641 = Wait Until Next ms Multiple(millisecond multiple=u32 300) -> ()  [unwired: 1 out]
    n13642 = Or(x="transfer atm", y="transfer atm auto") -> (x .or. y?=w18630:bool)
    n13643 = Or(x="transfer vacuum", y="transfer vacuum auto") -> (x .or. y?=w18629:bool)
    n13644 = Build Array(FALSE, w18630, w18629) -> (w18637:bool[])
    n13645 = Boolean Array To Number(Boolean array=w18637) -> (number=w18638:u32)
    n13646 = Mantissa & Exponent(0:w18638) -> (2:w18635:dbl)  [unwired: 1 out]
    n13647 = case shown="1" w18635 {
      frame 0, Default {
      }
      frame 1 {
        n13648 = local read "transfer atm"() -> (w18959:bool)
        n13649 = case shown="True" w18959 {
          tunnel: [TRUE ("T button?") w18963] -> w18958
          frame False {
            n13650 = local write "transfer atm auto"(FALSE ("transfer atm auto")) -> ()
          }
          frame True {
            n13651 = Two Button Dialog(message="Start Transfering at Atmosphere? ", 1:"No, Cancel" ("F button name (\"Cancel\")"), 2:"Yes, Continue" ("T button name (\"OK\")")) -> (T button?=w18963:bool)
            n13652 = local write "transfer atm"(FALSE ("transfer atm")) -> ()
          }
        }
        "TRNS atm alg" <- w18958
      }
      frame 2 {
        n13653 = local read "transfer vacuum"() -> (w18968:bool)
        n13654 = case shown="False" w18968 {
          tunnel: [TRUE ("T button?") w18972] -> w18967
          frame False {
            n13655 = local write "transfer vacuum auto"(FALSE ("transfer vacuum auto")) -> ()
          }
          frame True {
            n13656 = Two Button Dialog(message="Start Transfering under Vacuum ? ", 1:"No, Cancel" ("F button name (\"Cancel\")"), 2:"Yes, Continue" ("T button name (\"OK\")")) -> (T button?=w18972:bool)
            n13657 = local write "transfer vacuum"(FALSE ("transfer vacuum")) -> ()
          }
        }
        "TRNS vacuum alg" <- w18967
      }
    }
    n13658 = local read "TRNS vacuum alg"() -> (w18610:bool)